vi "CRYO_MASTER_temp_0911.vi"() -> ()   [LabVIEW 2017]
uses:
  LSI218Data.lvclass
  LSI336Data.lvclass
  USBData.lvclass
  6240AData.lvclass
  <vilib>/Analysis/3filter.llb/FIR Filter (DBL).vi
  <vilib>/DAQmx/create/channels.llb/DAQmx Create Channel (DO-Digital Output).vi
  <vilib>/DAQmx/miscellaneous.llb/DAQmx Fill In Error Info.vi
  <vilib>/DAQmx/create/channels.llb/DAQmx Create Channel (AO-Voltage-Basic).vi
  <vilib>/Analysis/NI_AALBase.lvlib
panel:
  in  "Record interval":i64=10
  out "Cycle #":u32=18
  in  "Measurement Interval (s)":dbl=1.0
  in  "Stop Button":bool
  in  "?":T1(tab)
  out "error out (USB6210/6218 AOUT)":errorcluster
  in  "AOUT 1 Label":string="KIKUSUI_I"
  in  "AOUT 0 Label":string="KIKUSUI_V"
  in  "DOUT Labels":string[](array[string])=["V1_NO", "V2_NC", "CV1"]
  in  "AOUT for Current CTRL":tag="Dev1/ao1"
  in  "AOUT For Voltage CTRL":tag="Dev1/ao0"
  out "AO task out":refnum<k21>="20200910_155539_AO"
  in  "Analog Out ON?":bool
  in  "InstName (USB6218)":string="USB6218"
  in  "USB6218 Config":T2(array[cluster])=[{"Label"="F_1", "FileFormat"="%5.5f", "Active?"=TRUE, "Physical CH"="Dev1/ai0", " terminal\n type"=10083, "ConversionType"={"Type"=enum."SimpleProp", "ConversionParameters"=[0.0, 5.0, 0.0, 500.0]}, "VoltageLimits"=[0.0, 5.0]}, {"Label"="F_2", "FileFormat"="%5.5f", "Active?"=TRUE, "Physical CH"="Dev1/ai1", " terminal\n type"=10083, "ConversionType"={"Type"=enum."SimpleProp", "ConversionParameters"=[0.0, 5.0, 0.0, 200.0]}, "VoltageLimits"=[0.0, 5.0]}, {"Label"="F_3", "FileFormat"="%5.5f", "Active?"=TRUE, "Physical CH"="Dev1/ai2", " terminal\n type"=10083, "ConversionType"={"Type"=enum."SimpleProp", "ConversionParameters"=[0.0, 5.0, 0.0, 200.0]}, "VoltageLimits"=[0.0, 5.0]}, {"Label"="F_4", "FileFormat"="%5.5f", "Active?"=TRUE, "Physical CH"="Dev1/ai3", " terminal\n type"=10083, "ConversionType"={"Type"=enum."SimpleProp", "ConversionParameters"=[0.0, 5.0, 0.0, 500.0]}, "VoltageLimits"=[0.0, 5.0]}, {"Label"="F_5", "FileFormat"="%5.5f", "Active?"=TRUE, "Physical CH"="Dev1/ai4", " terminal\n type"=10083, "ConversionType"={"Type"=enum."SimpleProp", "ConversionParameters"=[0.0, 5.0, 0.0, 500.0]}, "VoltageLimits"=[0.0, 5.0]}, {"Label"="I_CV", "FileFormat"="%3.5f", "Active?"=FALSE, "Physical CH"="Dev1/ai5", " terminal\n type"=10083, "ConversionType"={"Type"=enum."SimpleProp", "ConversionParameters"=[0.0, 5.0, 0.0, 2000.0]}, "VoltageLimits"=[0.0, 5.0]}, {"Label"="CV1_answer", "FileFormat"="%3.5f", "Active?"=FALSE, "Physical CH"="Dev1/ai6", " terminal\n type"=10083, "ConversionType"={"Type"=enum."Raw", "ConversionParameters"=[]}, "VoltageLimits"=[]}] {"terminal\n type" items=["Default"=-1, "RSE"=10083, "NRSE"=10078, "Differential"=10106, "Pseudodifferential"=12529]}
  out "error out (USB6218)":errorcluster={"status"=TRUE, "code"=-200489, "source"="DAQmx Create Channel (AI-Voltage-Basic).vi:1780001<append>\n<B>Channel Name: </B>Dev1/ai2\n\n<B>Task Name: </B>PreCooling_20200910_155626_USB6218__AIN"}
  out "error out (USB6210/6218 DOUT)":errorcluster
  out "Target Index":i32=6
  out "DOUT task out":refnum<k21>="20200910_155626_DO"
  in  "DOUT Physical CH":tag[](array[tag])=["Dev1/port1/line0", "Dev1/port1/line1", "Dev1/port1/line2"]
  in  "Dewar Regularization \nTarget Signal Label":string="P_Dewar"
  in  "Digital Out ON?":bool=TRUE
  in  "USB6210 Config":T2(array[cluster])=[{"Label"="P_ins", "FileFormat"="%5.5e", "Active?"=TRUE, "Physical CH"="Dev2/ai0", " terminal\n type"=10083, "ConversionType"={"Type"=enum."CC-10_LOG", "ConversionParameters"=[0.5, 9.0, 0.0, 1.0]}, "VoltageLimits"=[0.0, 10.0]}, {"Label"="P_4Kres", "FileFormat"="%5.5e", "Active?"=TRUE, "Physical CH"="Dev2/ai1", " terminal\n type"=10083, "ConversionType"={"Type"=enum."SimpleProp", "ConversionParameters"=[1.0, 5.0, 0.0, 200000.0]}, "VoltageLimits"=[0.0, 5.0]}, {"Label"="P_3HeIN", "FileFormat"="%5.5e", "Active?"=TRUE, "Physical CH"="Dev2/ai2", " terminal\n type"=10083, "ConversionType"={"Type"=enum."SimpleProp", "ConversionParameters"=[1.0, 5.0, 0.0, 200000.0]}, "VoltageLimits"=[0.0, 5.0]}, {"Label"="P_SldRTN", "FileFormat"="%5.5e", "Active?"=TRUE, "Physical CH"="Dev2/ai3", " terminal\n type"=10083, "ConversionType"={"Type"=enum."SimpleProp", "ConversionParameters"=[1.0, 5.0, 0.0, 200000.0]}, "VoltageLimits"=[0.0, 5.0]}, {"Label"="P_3Hepot", "FileFormat"="%5.5e", "Active?"=TRUE, "Physical CH"="Dev2/ai4", " terminal\n type"=10083, "ConversionType"={"Type"=enum."SimpleProp", "ConversionParameters"=[0.0, 10.0, 0.0, 133320.0]}, "VoltageLimits"=[0.0, 10.0]}, {"Label"="P_1Kpot", "FileFormat"="%5.5e", "Active?"=TRUE, "Physical CH"="Dev2/ai5", " terminal\n type"=10083, "ConversionType"={"Type"=enum."SimpleProp", "ConversionParameters"=[0.0, 10.0, 0.0, 133320.0]}, "VoltageLimits"=[0.0, 10.0]}, {"Label"="P_Dewar", "FileFormat"="%5.5e", "Active?"=TRUE, "Physical CH"="Dev2/ai6", " terminal\n type"=10083, "ConversionType"={"Type"=enum."SimpleProp", "ConversionParameters"=[1.0, 5.0, 0.0, 200000.0]}, "VoltageLimits"=[0.0, 5.0]}, {"Label"="DP_HEX4", "FileFormat"="%5.5e", "Active?"=TRUE, "Physical CH"="Dev2/ai7", " terminal\n type"=10083, "ConversionType"={"Type"=enum."SimpleProp", "ConversionParameters"=[1.0, 5.0, 0.0, 1000.0]}, "VoltageLimits"=[0.0, 5.0]}, {"Label"="DP_HEX5", "FileFormat"="%5.5e", "Active?"=TRUE, "Physical CH"="Dev2/ai8", " terminal\n type"=10083, "ConversionType"={"Type"=enum."SimpleProp", "ConversionParameters"=[1.0, 5.0, 0.0, 20000.0]}, "VoltageLimits"=[0.0, 5.0]}, {"Label"="L1", "FileFormat"="%5.5f", "Active?"=TRUE, "Physical CH"="Dev2/ai9", " terminal\n type"=10083, "ConversionType"={"Type"=enum."SimpleProp", "ConversionParameters"=[0.0, 10.0, 0.0, 100.0]}, "VoltageLimits"=[0.0, 10.0]}, {"Label"="L2-1", "FileFormat"="%5.5f", "Active?"=TRUE, "Physical CH"="Dev2/ai10", " terminal\n type"=10083, "ConversionType"={"Type"=enum."SimpleProp", "ConversionParameters"=[0.0, 10.0, 0.0, 100.0]}, "VoltageLimits"=[0.0, 10.0]}, {"Label"="L2-2", "FileFormat"="%5.5f", "Active?"=TRUE, "Physical CH"="Dev2/ai11", " terminal\n type"=10083, "ConversionType"={"Type"=enum."SimpleProp", "ConversionParameters"=[0.0, 10.0, 0.0, 100.0]}, "VoltageLimits"=[0.0, 10.0]}, {"Label"="L3", "FileFormat"="%5.5f", "Active?"=TRUE, "Physical CH"="Dev2/ai12", " terminal\n type"=10083, "ConversionType"={"Type"=enum."SimpleProp", "ConversionParameters"=[0.0, 10.0, 0.0, 100.0]}, "VoltageLimits"=[0.0, 10.0]}] {"terminal\n type" items=["Default"=-1, "RSE"=10083, "NRSE"=10078, "Differential"=10106, "Pseudodifferential"=12529]}
  in  "RUN identifier":string="PreCooling"
  in  "Base Path":path=path "C:/LabVIEW/DATA/Precooling"
  in  "InstName (USB6210)":string="USB6210"
  out "error out (USB6210)":errorcluster
  out "File Refn USB AO":refnum<file>
  out "File Refn USB DO":refnum<file>
  out "error out (LSI336)":errorcluster
  in  "InstName (LSI336)":string="LSI336"
  in  "FileFormat (336)":string="%4.4f"
  in  "LSI336Settings(X,Y)":T3(array[cluster])=[{"LSIName"="LSi336X", "Labels"=["T1K3-1", "T1K3-2", "T3He5", "T3He8"], "SensorLocations"=[enum."T1K3-1", enum."T1K3-2", enum."T3He5", enum."T3He8"], "Active?"=TRUE, "VISA res. name"="GPIB0::6::INSTR"}, {"LSIName"="LSi336Y", "Labels"=["T3He6-1", "T3He6-2", "T3He7-1", "T3He7-2"], "SensorLocations"=[enum."T3He6-1", enum."T3He6-2", enum."T3He7-1", enum."T3He7-2"], "Active?"=TRUE, "VISA res. name"="GPIB0::2::INSTR"}]
  in  "FileFormat (218)":string="%4.4f"
  in  "InstName (LSI218)":string="LSI218"
  in  "LSI218Settings(A-F)":T3(array[cluster])=[{"LSIName"="LSI218A", "Labels"=["T3He10", "T3He1-1", "TTH3", "TTH4", "TTH1", "TTH2", "T4He1", "T1K1"], "SensorLocations"=[enum."T3He10", enum."T3He1-1", enum."TTH3", enum."TTH4", enum."TTH1", enum."TTH2", enum."T4He1", enum."T1K1"], "Active?"=TRUE, "VISA res. name"="GPIB0::7::INSTR"}, {"LSIName"="LSI218B", "Labels"=["N.C.", "N.C.", "N.C.", "N.C.", "T3He2-1", "T3He2-2", "T3He3", "T3He1-4"], "SensorLocations"=[enum."N.C.", enum."N.C.", enum."N.C.", enum."T3He1-4", enum."T3He2-1", enum."T3He2-2", enum."T3He3", enum."T3He1-4"], "Active?"=TRUE, "VISA res. name"="GPIB0::4::INSTR"}, {"LSIName"="LSI218C", "Labels"=["T4He3-1", "T4He3-2", "T4He3-3", "T4He3-4", "T4He2-1", "T4He2-2", "T4He4", "T4He5"], "SensorLocations"=[enum."T4He3-1", enum."T4He3-2", enum."T4He3-3", enum."T4He3-4", enum."T4He2-1", enum."T4He2-2", enum."T4He4", enum."T4He5"], "Active?"=TRUE, "VISA res. name"="GPIB0::3::INSTR"}, {"LSIName"="LSI218D", "Labels"=["T4He6", "T4He9", "T3He1-2", "T3He1-3", "T4He7", "T4He8", "T4He10", "T1K6"], "SensorLocations"=[enum."T4He6", enum."T4He9", enum."T3He1-2", enum."T3He1-3", enum."T4He7", enum."T4He8", enum."T4He10", enum."T1K6"], "Active?"=TRUE, "VISA res. name"="GPIB0::5::INSTR"}, {"LSIName"="LSI218E", "Labels"=["TIP1", "N.C.", "TIP2", "N.C.", "TIP3", "TIP4", "TIP5", "N.C."], "SensorLocations"=[enum."TIP1", enum."N.C.", enum."TIP2", enum."N.C.", enum."TIP3", enum."TIP4", enum."TIP5", enum."N.C."], "Active?"=TRUE, "VISA res. name"="GPIB0::11::INSTR"}, {"LSIName"="LSI218F", "Labels"=["T1K2", "T1K4", "T1K5", "T3He4", "T3He9", "TIP6", "N.C.", "N.C."], "SensorLocations"=[enum."T1K2", enum."T1K4", enum."T1K5", enum."T3He4", enum."T3He9", enum."TIP6", enum."N.C.", enum."N.C."], "Active?"=TRUE, "VISA res. name"="GPIB0::8::INSTR"}]
  out "error out (LSI218)":errorcluster
  in  "FIle suffix 4":string="Graph4"
  in  "Take Screenshot! 4":bool
  in  "FIle suffix 3":string="Graph3"
  in  "Take Screenshot! 3":bool
  in  "FIle suffix 2":string="Graph2"
  in  "Take Screenshot! 2":bool
  in  "FIle suffix 1":string="Graph1"
  in  "Take Screenshot! 1":bool
  in  "log/linear 2":bool
  in  "Tab Control 2":T4(tab)=enum."USB6218"
  in  "Plot selecter (USB6210)\n    1      2     3     4":bool[][](array[boolean])=[[FALSE, FALSE, TRUE, FALSE], [FALSE, FALSE, TRUE, FALSE], [FALSE, FALSE, TRUE, FALSE], [FALSE, FALSE, TRUE, FALSE], [FALSE, FALSE, TRUE, FALSE], [FALSE, FALSE, TRUE, FALSE], [TRUE, FALSE, FALSE, FALSE], [FALSE, FALSE, TRUE, FALSE], [FALSE, FALSE, TRUE, FALSE], [FALSE, FALSE, FALSE, TRUE], [FALSE, FALSE, FALSE, TRUE], [FALSE, FALSE, FALSE, TRUE], [FALSE, FALSE, FALSE, TRUE], [FALSE, FALSE, FALSE, FALSE], [FALSE, FALSE, FALSE, FALSE], [FALSE, FALSE, FALSE, FALSE]]
  out "All Labels (USB6210)":string[](array[string])=["P_ins", "P_4Kres", "P_3HeIN", "P_SldRTN", "P_3Hepot", "P_1Kpot", "P_Dewar", "DP_HEX4", "DP_HEX5", "L1", "L2-1", "L2-2", "L3"]
  out "Last Data \n(USB6210)":dbl[](array[numeric])=[0.0009060437653636275, 100884.97913376133, 100585.6935800327, 100396.58457551748, 100537.343311204, 100655.70674054678, 101557.55033670987, -10.021506447432133, 71.06102831736294, 100.09004251119043, 0.10469622427214367, 0.11521822711602545, 99.57181211647702] format="%#_6e"
  out "Time of Last Measurement (USB6210)":timestamp=timestamp(3682565805.197301 s since 1904-01-01)
  out "USB6210 Status":T5(ring)=enum."Ready"
  out "Last Vol\n(USB6210)":dbl[](array[numeric])=[5.978574588130271, 3.0176995826752266, 3.011713871600654, 3.0079316915103496, 7.541054853825682, 7.549932998840893, 3.0311510067341976, 0.9599139742102715, 1.0142122056634726, 10.009004251119043, 0.010469622427214368, 0.011521822711602545, 9.957181211647702] format="%_5f"
  out "Time of Last Measurement (USB6218)":timestamp
  out "USB6218 Status":T5(ring)=enum."Ready"
  out "Last Vol \n(USB6218)":dbl[](array[numeric]) format="%_5f"
  out "Last Data \n(USB6218)":dbl[](array[numeric]) format="%#_6e"
  out "All Labels (USB6218)":string[](array[string])
  in  "Plot selecter (USB6218)\n    1      2     3     4":bool[][](array[boolean])=[[FALSE, FALSE, TRUE, FALSE], [FALSE, FALSE, TRUE, FALSE], [FALSE, FALSE, TRUE, FALSE], [FALSE, FALSE, TRUE, FALSE], [FALSE, FALSE, TRUE, FALSE], [FALSE, FALSE, TRUE, FALSE], [TRUE, FALSE, FALSE, FALSE], [FALSE, FALSE, TRUE, FALSE], [FALSE, FALSE, TRUE, FALSE], [FALSE, FALSE, FALSE, TRUE], [FALSE, FALSE, FALSE, TRUE], [FALSE, FALSE, FALSE, TRUE], [FALSE, FALSE, FALSE, TRUE], [FALSE, FALSE, FALSE, FALSE], [FALSE, FALSE, FALSE, FALSE], [FALSE, FALSE, FALSE, FALSE]]
  out "Time of Last Measurement (LSI218)":timestamp=timestamp(3682565805.197301 s since 1904-01-01)
  out "LSI218 Status":T6(ring)=enum."Measuring"
  out "Last Data \nLSI218 (1)":dbl[](array[numeric])=[297.63, 297.76, 296.71, 297.24, 295.38, 295.52, 294.91, 295.07, 30.0, 0.0, 0.0, 0.0, 296.58, 296.99, 295.68, 297.19, 297.39, 297.55, 297.28, 297.31, 296.61, 296.28, 296.32, 296.17]
  out "Labels LSI218 (1)":string[](array[string])=["T3He10", "T3He1-1", "TTH3", "TTH4", "TTH1", "TTH2", "T4He1", "T1K1", "N.C.", "N.C.", "N.C.", "N.C.", "T3He2-1", "T3He2-2", "T3He3", "T3He1-4", "T4He3-1", "T4He3-2", "T4He3-3", "T4He3-4", "T4He2-1", "T4He2-2", "T4He4", "T4He5"]
  in  "Plot selecter LSI218(1)\n    1      2     3     4":bool[][](array[boolean])=[[FALSE, FALSE, FALSE, FALSE], [FALSE, FALSE, FALSE, FALSE], [FALSE, FALSE, FALSE, FALSE], [FALSE, FALSE, FALSE, FALSE], [FALSE, FALSE, FALSE, FALSE], [FALSE, FALSE, FALSE, FALSE], [FALSE, FALSE, FALSE, FALSE], [FALSE, FALSE, FALSE, FALSE], [FALSE, FALSE, FALSE, FALSE], [FALSE, FALSE, FALSE, FALSE], [FALSE, FALSE, FALSE, FALSE], [FALSE, FALSE, FALSE, FALSE], [FALSE, FALSE, FALSE, FALSE], [FALSE, FALSE, FALSE, FALSE], [FALSE, FALSE, FALSE, FALSE], [FALSE, FALSE, FALSE, FALSE], [FALSE, FALSE, FALSE, FALSE], [FALSE, FALSE, FALSE, FALSE], [FALSE, FALSE, FALSE, FALSE], [FALSE, FALSE, FALSE, FALSE], [FALSE, FALSE, FALSE, FALSE], [FALSE, FALSE, FALSE, FALSE], [FALSE, FALSE, FALSE, FALSE], [FALSE, FALSE, FALSE, FALSE]]
  out "Active?\n (1)":bool[](array[boolean])=[TRUE, TRUE, TRUE, TRUE, TRUE, TRUE, TRUE, TRUE, TRUE, TRUE, TRUE, TRUE, TRUE, TRUE, TRUE, TRUE, TRUE, TRUE, TRUE, TRUE, TRUE, TRUE, TRUE, TRUE]
  out "Labels LSI218 (2)":string[](array[string])=["T4He6", "T4He9", "T3He1-2", "T3He1-3", "T4He7", "T4He8", "T4He10", "T1K6", "TIP1", "N.C.", "TIP2", "N.C.", "TIP3", "TIP4", "TIP5", "N.C.", "T1K2", "T1K4", "T1K5", "T3He4", "T3He9", "TIP6", "N.C.", "N.C."]
  out "Active?\n(2)":bool[](array[boolean])=[TRUE, TRUE, TRUE, TRUE, TRUE, TRUE, TRUE, TRUE, TRUE, TRUE, TRUE, TRUE, TRUE, TRUE, TRUE, TRUE, TRUE, TRUE, TRUE, TRUE, TRUE, TRUE, TRUE, TRUE]
  out "Last Data \nLSI218 (2)":dbl[](array[numeric])=[296.4, 297.17, 297.92, 297.51, 296.71, 297.02, 296.96, 297.42, 296.77, 0.0, 296.31, 688.49, 296.06, 295.63, 295.73, 688.58, 302.11, 301.08, 296.91, 291.77, 288.69, 280.14, 0.433, 0.0]
  in  "Plot selecter LSI218(2)\n    1      2     3     4":bool[][](array[boolean])=[[FALSE, TRUE, FALSE, FALSE], [FALSE, TRUE, FALSE, FALSE], [FALSE, TRUE, FALSE, FALSE], [FALSE, TRUE, FALSE, FALSE], [FALSE, TRUE, FALSE, FALSE], [FALSE, TRUE, FALSE, FALSE], [FALSE, TRUE, FALSE, FALSE], [FALSE, TRUE, FALSE, FALSE], [FALSE, TRUE, FALSE, FALSE], [FALSE, TRUE, FALSE, FALSE], [FALSE, TRUE, FALSE, FALSE], [FALSE, FALSE, FALSE, FALSE], [FALSE, FALSE, FALSE, FALSE], [FALSE, FALSE, FALSE, FALSE], [FALSE, FALSE, FALSE, FALSE], [FALSE, FALSE, FALSE, FALSE], [FALSE, FALSE, FALSE, FALSE], [FALSE, FALSE, FALSE, FALSE], [FALSE, FALSE, FALSE, FALSE], [FALSE, FALSE, FALSE, FALSE], [FALSE, FALSE, FALSE, FALSE], [FALSE, FALSE, FALSE, FALSE], [FALSE, FALSE, FALSE, FALSE], [FALSE, FALSE, FALSE, FALSE]]
  in  "Plot selecter LSI336 \n     1      2     3     4":bool[][](array[boolean])=[[FALSE, TRUE, FALSE, FALSE], [FALSE, TRUE, FALSE, FALSE], [FALSE, TRUE, FALSE, FALSE], [FALSE, TRUE, FALSE, FALSE], [FALSE, TRUE, FALSE, FALSE], [FALSE, TRUE, FALSE, FALSE], [FALSE, TRUE, FALSE, FALSE], [FALSE, TRUE, FALSE, FALSE]]
  out "Time of Last Measurement (LSI336) 2":timestamp=timestamp(3682565805.197301 s since 1904-01-01)
  out "Last Data \nLSI336":dbl[](array[numeric])=[296.838, 296.434, 296.022, 296.217, 295.887, 295.842, 295.916, 296.504]
  out "Active?\n(LSI336)":bool[](array[boolean])=[TRUE, TRUE, TRUE, TRUE, TRUE, TRUE, TRUE, TRUE]
  out "Labels LSI336":string[](array[string])=["T1K3-1", "T1K3-2", "T3He5", "T3He8", "T3He6-1", "T3He6-2", "T3He7-1", "T3He7-2"]
  out "LSI336 Status":T6(ring)=enum."Measuring"
  out "Graph 1":T7(graph)=[{"TimeArray"=[timestamp(3682565788.1889906 s since 1904-01-01), timestamp(3682565789.190164 s since 1904-01-01), timestamp(3682565790.191844 s since 1904-01-01), timestamp(3682565791.191016 s since 1904-01-01), timestamp(3682565792.191493 s since 1904-01-01), timestamp(3682565793.190962 s since 1904-01-01), timestamp(3682565794.192923 s since 1904-01-01), timestamp(3682565795.1943216 s since 1904-01-01), timestamp(3682565796.1945167 s since 1904-01-01), timestamp(3682565797.194023 s since 1904-01-01), timestamp(3682565798.195678 s since 1904-01-01), timestamp(3682565799.194545 s since 1904-01-01), timestamp(3682565800.194017 s since 1904-01-01), timestamp(3682565801.196416 s since 1904-01-01), timestamp(3682565802.1962314 s since 1904-01-01), timestamp(3682565803.1960993 s since 1904-01-01), timestamp(3682565804.196091 s since 1904-01-01), timestamp(3682565805.197301 s since 1904-01-01)], "LDArray"=[98878.77979362432]}] caption="XY Graph"
  in  "log/linear 1":bool
  out "Graph 2":T8(graph)=[{"TimeArray"=[timestamp(3682565788.1889906 s since 1904-01-01), timestamp(3682565789.190164 s since 1904-01-01), timestamp(3682565790.191844 s since 1904-01-01), timestamp(3682565791.191016 s since 1904-01-01), timestamp(3682565792.191493 s since 1904-01-01), timestamp(3682565793.190962 s since 1904-01-01), timestamp(3682565794.192923 s since 1904-01-01), timestamp(3682565795.1943216 s since 1904-01-01), timestamp(3682565796.1945167 s since 1904-01-01), timestamp(3682565797.194023 s since 1904-01-01), timestamp(3682565798.1947985 s since 1904-01-01), timestamp(3682565799.194545 s since 1904-01-01), timestamp(3682565800.194017 s since 1904-01-01), timestamp(3682565801.1955366 s since 1904-01-01), timestamp(3682565802.1962314 s since 1904-01-01), timestamp(3682565803.1960993 s since 1904-01-01), timestamp(3682565804.196091 s since 1904-01-01), timestamp(3682565805.197301 s since 1904-01-01)], "DataArray"=[296.44, 296.4, 296.4, 296.4, 296.43, 296.43, 296.39, 296.41, 296.43, 296.4, 296.39, 296.41, 296.38, 296.38, 296.41, 296.42, 296.41, 296.4]}, {"TimeArray"=[timestamp(3682565788.1889906 s since 1904-01-01), timestamp(3682565789.190164 s since 1904-01-01), timestamp(3682565790.191844 s since 1904-01-01), timestamp(3682565791.191016 s since 1904-01-01), timestamp(3682565792.191493 s since 1904-01-01), timestamp(3682565793.190962 s since 1904-01-01), timestamp(3682565794.192923 s since 1904-01-01), timestamp(3682565795.1943216 s since 1904-01-01), timestamp(3682565796.1945167 s since 1904-01-01), timestamp(3682565797.194023 s since 1904-01-01), timestamp(3682565798.1947985 s since 1904-01-01), timestamp(3682565799.194545 s since 1904-01-01), timestamp(3682565800.194017 s since 1904-01-01), timestamp(3682565801.1955366 s since 1904-01-01), timestamp(3682565802.1962314 s since 1904-01-01), timestamp(3682565803.1960993 s since 1904-01-01), timestamp(3682565804.196091 s since 1904-01-01), timestamp(3682565805.197301 s since 1904-01-01)], "DataArray"=[297.15, 297.15, 297.15, 297.15, 297.16, 297.16, 297.14, 297.14, 297.15, 297.13, 297.16, 297.14, 297.14, 297.14, 297.12, 297.14, 297.14, 297.17]}, {"TimeArray"=[timestamp(3682565788.1889906 s since 1904-01-01), timestamp(3682565789.190164 s since 1904-01-01), timestamp(3682565790.191844 s since 1904-01-01), timestamp(3682565791.191016 s since 1904-01-01), timestamp(3682565792.191493 s since 1904-01-01), timestamp(3682565793.190962 s since 1904-01-01), timestamp(3682565794.192923 s since 1904-01-01), timestamp(3682565795.1943216 s since 1904-01-01), timestamp(3682565796.1945167 s since 1904-01-01), timestamp(3682565797.194023 s since 1904-01-01), timestamp(3682565798.1947985 s since 1904-01-01), timestamp(3682565799.194545 s since 1904-01-01), timestamp(3682565800.194017 s since 1904-01-01), timestamp(3682565801.1955366 s since 1904-01-01), timestamp(3682565802.1962314 s since 1904-01-01), timestamp(3682565803.1960993 s since 1904-01-01), timestamp(3682565804.196091 s since 1904-01-01), timestamp(3682565805.197301 s since 1904-01-01)], "DataArray"=[297.94, 297.93, 297.96, 297.92, 297.94, 297.93, 297.93, 297.93, 297.93, 297.94, 297.96, 297.93, 297.93, 297.94, 297.93, 297.93, 297.93, 297.92]}, {"TimeArray"=[timestamp(3682565788.1889906 s since 1904-01-01), timestamp(3682565789.190164 s since 1904-01-01), timestamp(3682565790.191844 s since 1904-01-01), timestamp(3682565791.191016 s since 1904-01-01), timestamp(3682565792.191493 s since 1904-01-01), timestamp(3682565793.190962 s since 1904-01-01), timestamp(3682565794.192923 s since 1904-01-01), timestamp(3682565795.1943216 s since 1904-01-01), timestamp(3682565796.1945167 s since 1904-01-01), timestamp(3682565797.194023 s since 1904-01-01), timestamp(3682565798.1947985 s since 1904-01-01), timestamp(3682565799.194545 s since 1904-01-01), timestamp(3682565800.194017 s since 1904-01-01), timestamp(3682565801.1955366 s since 1904-01-01), timestamp(3682565802.1962314 s since 1904-01-01), timestamp(3682565803.1960993 s since 1904-01-01), timestamp(3682565804.196091 s since 1904-01-01), timestamp(3682565805.197301 s since 1904-01-01)], "DataArray"=[297.53, 297.5, 297.52, 297.51, 297.52, 297.52, 297.54, 297.54, 297.53, 297.51, 297.52, 297.52, 297.53, 297.52, 297.53, 297.52, 297.53, 297.51]}, {"TimeArray"=[timestamp(3682565788.1889906 s since 1904-01-01), timestamp(3682565789.190164 s since 1904-01-01), timestamp(3682565790.191844 s since 1904-01-01), timestamp(3682565791.191016 s since 1904-01-01), timestamp(3682565792.191493 s since 1904-01-01), timestamp(3682565793.190962 s since 1904-01-01), timestamp(3682565794.192923 s since 1904-01-01), timestamp(3682565795.1943216 s since 1904-01-01), timestamp(3682565796.1945167 s since 1904-01-01), timestamp(3682565797.194023 s since 1904-01-01), timestamp(3682565798.1947985 s since 1904-01-01), timestamp(3682565799.194545 s since 1904-01-01), timestamp(3682565800.194017 s since 1904-01-01), timestamp(3682565801.1955366 s since 1904-01-01), timestamp(3682565802.1962314 s since 1904-01-01), timestamp(3682565803.1960993 s since 1904-01-01), timestamp(3682565804.196091 s since 1904-01-01), timestamp(3682565805.197301 s since 1904-01-01)], "DataArray"=[296.7, 296.71, 296.71, 296.72, 296.7, 296.69, 296.7, 296.69, 296.7, 296.7, 296.7, 296.7, 296.71, 296.7, 296.71, 296.68, 296.7, 296.71]}, {"TimeArray"=[timestamp(3682565788.1889906 s since 1904-01-01), timestamp(3682565789.190164 s since 1904-01-01), timestamp(3682565790.191844 s since 1904-01-01), timestamp(3682565791.191016 s since 1904-01-01), timestamp(3682565792.191493 s since 1904-01-01), timestamp(3682565793.190962 s since 1904-01-01), timestamp(3682565794.192923 s since 1904-01-01), timestamp(3682565795.1943216 s since 1904-01-01), timestamp(3682565796.1945167 s since 1904-01-01), timestamp(3682565797.194023 s since 1904-01-01), timestamp(3682565798.1947985 s since 1904-01-01), timestamp(3682565799.194545 s since 1904-01-01), timestamp(3682565800.194017 s since 1904-01-01), timestamp(3682565801.1955366 s since 1904-01-01), timestamp(3682565802.1962314 s since 1904-01-01), timestamp(3682565803.1960993 s since 1904-01-01), timestamp(3682565804.196091 s since 1904-01-01), timestamp(3682565805.197301 s since 1904-01-01)], "DataArray"=[297.02, 297.03, 297.04, 297.03, 297.0, 297.02, 297.0, 297.02, 297.05, 297.0, 297.0, 297.0, 297.01, 297.02, 297.03, 297.0, 297.02, 297.02]}, {"TimeArray"=[timestamp(3682565788.1889906 s since 1904-01-01), timestamp(3682565789.190164 s since 1904-01-01), timestamp(3682565790.191844 s since 1904-01-01), timestamp(3682565791.191016 s since 1904-01-01), timestamp(3682565792.191493 s since 1904-01-01), timestamp(3682565793.190962 s since 1904-01-01), timestamp(3682565794.192923 s since 1904-01-01), timestamp(3682565795.1943216 s since 1904-01-01), timestamp(3682565796.1945167 s since 1904-01-01), timestamp(3682565797.194023 s since 1904-01-01), timestamp(3682565798.1947985 s since 1904-01-01), timestamp(3682565799.194545 s since 1904-01-01), timestamp(3682565800.194017 s since 1904-01-01), timestamp(3682565801.1955366 s since 1904-01-01), timestamp(3682565802.1962314 s since 1904-01-01), timestamp(3682565803.1960993 s since 1904-01-01), timestamp(3682565804.196091 s since 1904-01-01), timestamp(3682565805.197301 s since 1904-01-01)], "DataArray"=[296.96, 296.97, 296.96, 296.98, 296.96, 296.95, 296.98, 296.99, 296.97, 296.96, 296.95, 296.94, 296.95, 296.95, 296.97, 296.95, 296.96, 296.96]}, {"TimeArray"=[timestamp(3682565788.1889906 s since 1904-01-01), timestamp(3682565789.190164 s since 1904-01-01), timestamp(3682565790.191844 s since 1904-01-01), timestamp(3682565791.191016 s since 1904-01-01), timestamp(3682565792.191493 s since 1904-01-01), timestamp(3682565793.190962 s since 1904-01-01), timestamp(3682565794.192923 s since 1904-01-01), timestamp(3682565795.1943216 s since 1904-01-01), timestamp(3682565796.1945167 s since 1904-01-01), timestamp(3682565797.194023 s since 1904-01-01), timestamp(3682565798.1947985 s since 1904-01-01), timestamp(3682565799.194545 s since 1904-01-01), timestamp(3682565800.194017 s since 1904-01-01), timestamp(3682565801.1955366 s since 1904-01-01), timestamp(3682565802.1962314 s since 1904-01-01), timestamp(3682565803.1960993 s since 1904-01-01), timestamp(3682565804.196091 s since 1904-01-01), timestamp(3682565805.197301 s since 1904-01-01)], "DataArray"=[297.4, 297.41, 297.4, 297.4, 297.41, 297.42, 297.41, 297.42, 297.41, 297.4, 297.42, 297.41, 297.42, 297.39, 297.42, 297.4, 297.42, 297.42]}, {"TimeArray"=[timestamp(3682565788.1889906 s since 1904-01-01), timestamp(3682565789.190164 s since 1904-01-01), timestamp(3682565790.191844 s since 1904-01-01), timestamp(3682565791.191016 s since 1904-01-01), timestamp(3682565792.191493 s since 1904-01-01), timestamp(3682565793.190962 s since 1904-01-01), timestamp(3682565794.192923 s since 1904-01-01), timestamp(3682565795.1943216 s since 1904-01-01), timestamp(3682565796.1945167 s since 1904-01-01), timestamp(3682565797.194023 s since 1904-01-01), timestamp(3682565798.1947985 s since 1904-01-01), timestamp(3682565799.194545 s since 1904-01-01), timestamp(3682565800.194017 s since 1904-01-01), timestamp(3682565801.1955366 s since 1904-01-01), timestamp(3682565802.1962314 s since 1904-01-01), timestamp(3682565803.1960993 s since 1904-01-01), timestamp(3682565804.196091 s since 1904-01-01), timestamp(3682565805.197301 s since 1904-01-01)], "DataArray"=[296.76, 296.76, 296.76, 296.76, 296.76, 296.77, 296.76, 296.77, 296.76, 296.76, 296.76, 296.76, 296.76, 296.76, 296.76, 296.76, 296.77, 296.77]}, {"TimeArray"=[timestamp(3682565788.1889906 s since 1904-01-01), timestamp(3682565789.190164 s since 1904-01-01), timestamp(3682565790.191844 s since 1904-01-01), timestamp(3682565791.191016 s since 1904-01-01), timestamp(3682565792.191493 s since 1904-01-01), timestamp(3682565793.190962 s since 1904-01-01), timestamp(3682565794.192923 s since 1904-01-01), timestamp(3682565795.1943216 s since 1904-01-01), timestamp(3682565796.1945167 s since 1904-01-01), timestamp(3682565797.194023 s since 1904-01-01), timestamp(3682565798.1947985 s since 1904-01-01), timestamp(3682565799.194545 s since 1904-01-01), timestamp(3682565800.194017 s since 1904-01-01), timestamp(3682565801.1955366 s since 1904-01-01), timestamp(3682565802.1962314 s since 1904-01-01), timestamp(3682565803.1960993 s since 1904-01-01), timestamp(3682565804.196091 s since 1904-01-01), timestamp(3682565805.197301 s since 1904-01-01)], "DataArray"=[0.0, 0.0, 0.0, 0.0, 0.0, 0.0, 0.0, 0.0, 0.0, 0.0, 0.0, 0.0, 0.0, 0.0, 0.0, 0.0, 0.0, 0.0]}, {"TimeArray"=[timestamp(3682565788.1889906 s since 1904-01-01), timestamp(3682565789.190164 s since 1904-01-01), timestamp(3682565790.191844 s since 1904-01-01), timestamp(3682565791.191016 s since 1904-01-01), timestamp(3682565792.191493 s since 1904-01-01), timestamp(3682565793.190962 s since 1904-01-01), timestamp(3682565794.192923 s since 1904-01-01), timestamp(3682565795.1943216 s since 1904-01-01), timestamp(3682565796.1945167 s since 1904-01-01), timestamp(3682565797.194023 s since 1904-01-01), timestamp(3682565798.1947985 s since 1904-01-01), timestamp(3682565799.194545 s since 1904-01-01), timestamp(3682565800.194017 s since 1904-01-01), timestamp(3682565801.1955366 s since 1904-01-01), timestamp(3682565802.1962314 s since 1904-01-01), timestamp(3682565803.1960993 s since 1904-01-01), timestamp(3682565804.196091 s since 1904-01-01), timestamp(3682565805.197301 s since 1904-01-01)], "DataArray"=[296.31, 296.33, 296.32, 296.31, 296.33, 296.32, 296.32, 296.32, 296.32, 296.32, 296.33, 296.33, 296.31, 296.32, 296.33, 296.31, 296.32, 296.31]}, {"TimeArray"=[timestamp(3682565788.1889906 s since 1904-01-01), timestamp(3682565789.190164 s since 1904-01-01), timestamp(3682565790.191844 s since 1904-01-01), timestamp(3682565791.191016 s since 1904-01-01), timestamp(3682565792.191493 s since 1904-01-01), timestamp(3682565793.190962 s since 1904-01-01), timestamp(3682565794.192923 s since 1904-01-01), timestamp(3682565795.1943216 s since 1904-01-01), timestamp(3682565796.1945167 s since 1904-01-01), timestamp(3682565797.194023 s since 1904-01-01), timestamp(3682565798.1947985 s since 1904-01-01), timestamp(3682565799.194545 s since 1904-01-01), timestamp(3682565800.194017 s since 1904-01-01), timestamp(3682565801.1955366 s since 1904-01-01), timestamp(3682565802.1962314 s since 1904-01-01), timestamp(3682565803.1960993 s since 1904-01-01), timestamp(3682565804.196091 s since 1904-01-01), timestamp(3682565805.197301 s since 1904-01-01)], "DataArray"=[296.847, 296.84, 296.846, 296.853, 296.853, 296.84, 296.845, 296.857, 296.848, 296.872, 296.855, 296.849, 296.848, 296.854, 296.853, 296.859, 296.85, 296.838]}, {"TimeArray"=[timestamp(3682565788.1889906 s since 1904-01-01), timestamp(3682565789.190164 s since 1904-01-01), timestamp(3682565790.191844 s since 1904-01-01), timestamp(3682565791.191016 s since 1904-01-01), timestamp(3682565792.191493 s since 1904-01-01), timestamp(3682565793.190962 s since 1904-01-01), timestamp(3682565794.192923 s since 1904-01-01), timestamp(3682565795.1943216 s since 1904-01-01), timestamp(3682565796.1945167 s since 1904-01-01), timestamp(3682565797.194023 s since 1904-01-01), timestamp(3682565798.1947985 s since 1904-01-01), timestamp(3682565799.194545 s since 1904-01-01), timestamp(3682565800.194017 s since 1904-01-01), timestamp(3682565801.1955366 s since 1904-01-01), timestamp(3682565802.1962314 s since 1904-01-01), timestamp(3682565803.1960993 s since 1904-01-01), timestamp(3682565804.196091 s since 1904-01-01), timestamp(3682565805.197301 s since 1904-01-01)], "DataArray"=[296.447, 296.444, 296.434, 296.439, 296.434, 296.44, 296.441, 296.446, 296.444, 296.461, 296.459, 296.445, 296.453, 296.446, 296.443, 296.445, 296.445, 296.434]}, {"TimeArray"=[timestamp(3682565788.1889906 s since 1904-01-01), timestamp(3682565789.190164 s since 1904-01-01), timestamp(3682565790.191844 s since 1904-01-01), timestamp(3682565791.191016 s since 1904-01-01), timestamp(3682565792.191493 s since 1904-01-01), timestamp(3682565793.190962 s since 1904-01-01), timestamp(3682565794.192923 s since 1904-01-01), timestamp(3682565795.1943216 s since 1904-01-01), timestamp(3682565796.1945167 s since 1904-01-01), timestamp(3682565797.194023 s since 1904-01-01), timestamp(3682565798.1947985 s since 1904-01-01), timestamp(3682565799.194545 s since 1904-01-01), timestamp(3682565800.194017 s since 1904-01-01), timestamp(3682565801.1955366 s since 1904-01-01), timestamp(3682565802.1962314 s since 1904-01-01), timestamp(3682565803.1960993 s since 1904-01-01), timestamp(3682565804.196091 s since 1904-01-01), timestamp(3682565805.197301 s since 1904-01-01)], "DataArray"=[296.043, 296.016, 296.025, 296.028, 296.025, 296.018, 296.021, 296.016, 296.018, 296.027, 296.024, 296.016, 296.024, 296.014, 296.023, 296.031, 296.013, 296.022]}, {"TimeArray"=[timestamp(3682565788.1889906 s since 1904-01-01), timestamp(3682565789.190164 s since 1904-01-01), timestamp(3682565790.191844 s since 1904-01-01), timestamp(3682565791.191016 s since 1904-01-01), timestamp(3682565792.191493 s since 1904-01-01), timestamp(3682565793.190962 s since 1904-01-01), timestamp(3682565794.192923 s since 1904-01-01), timestamp(3682565795.1943216 s since 1904-01-01), timestamp(3682565796.1945167 s since 1904-01-01), timestamp(3682565797.194023 s since 1904-01-01), timestamp(3682565798.1947985 s since 1904-01-01), timestamp(3682565799.194545 s since 1904-01-01), timestamp(3682565800.194017 s since 1904-01-01), timestamp(3682565801.1955366 s since 1904-01-01), timestamp(3682565802.1962314 s since 1904-01-01), timestamp(3682565803.1960993 s since 1904-01-01), timestamp(3682565804.196091 s since 1904-01-01), timestamp(3682565805.197301 s since 1904-01-01)], "DataArray"=[296.255, 296.223, 296.212, 296.217, 296.221, 296.211, 296.215, 296.214, 296.221, 296.222, 296.22, 296.22, 296.215, 296.21, 296.215, 296.221, 296.21, 296.217]}, {"TimeArray"=[timestamp(3682565788.1889906 s since 1904-01-01), timestamp(3682565789.190164 s since 1904-01-01), timestamp(3682565790.191844 s since 1904-01-01), timestamp(3682565791.191016 s since 1904-01-01), timestamp(3682565792.191493 s since 1904-01-01), timestamp(3682565793.190962 s since 1904-01-01), timestamp(3682565794.192923 s since 1904-01-01), timestamp(3682565795.1943216 s since 1904-01-01), timestamp(3682565796.1945167 s since 1904-01-01), timestamp(3682565797.194023 s since 1904-01-01), timestamp(3682565798.1947985 s since 1904-01-01), timestamp(3682565799.194545 s since 1904-01-01), timestamp(3682565800.194017 s since 1904-01-01), timestamp(3682565801.1955366 s since 1904-01-01), timestamp(3682565802.1962314 s since 1904-01-01), timestamp(3682565803.1960993 s since 1904-01-01), timestamp(3682565804.196091 s since 1904-01-01), timestamp(3682565805.197301 s since 1904-01-01)], "DataArray"=[295.89, 295.881, 295.884, 295.884, 295.892, 295.875, 295.898, 295.88, 295.894, 295.891, 295.897, 295.894, 295.896, 295.879, 295.893, 295.894, 295.892, 295.887]}, {"TimeArray"=[timestamp(3682565788.1889906 s since 1904-01-01), timestamp(3682565789.190164 s since 1904-01-01), timestamp(3682565790.191844 s since 1904-01-01), timestamp(3682565791.191016 s since 1904-01-01), timestamp(3682565792.191493 s since 1904-01-01), timestamp(3682565793.190962 s since 1904-01-01), timestamp(3682565794.192923 s since 1904-01-01), timestamp(3682565795.1943216 s since 1904-01-01), timestamp(3682565796.1945167 s since 1904-01-01), timestamp(3682565797.194023 s since 1904-01-01), timestamp(3682565798.1947985 s since 1904-01-01), timestamp(3682565799.194545 s since 1904-01-01), timestamp(3682565800.194017 s since 1904-01-01), timestamp(3682565801.1955366 s since 1904-01-01), timestamp(3682565802.1962314 s since 1904-01-01), timestamp(3682565803.1960993 s since 1904-01-01), timestamp(3682565804.196091 s since 1904-01-01), timestamp(3682565805.197301 s since 1904-01-01)], "DataArray"=[295.848, 295.843, 295.842, 295.856, 295.851, 295.842, 295.843, 295.849, 295.851, 295.846, 295.842, 295.842, 295.842, 295.854, 295.833, 295.844, 295.852, 295.842]}, {"TimeArray"=[timestamp(3682565788.1889906 s since 1904-01-01), timestamp(3682565789.190164 s since 1904-01-01), timestamp(3682565790.191844 s since 1904-01-01), timestamp(3682565791.191016 s since 1904-01-01), timestamp(3682565792.191493 s since 1904-01-01), timestamp(3682565793.190962 s since 1904-01-01), timestamp(3682565794.192923 s since 1904-01-01), timestamp(3682565795.1943216 s since 1904-01-01), timestamp(3682565796.1945167 s since 1904-01-01), timestamp(3682565797.194023 s since 1904-01-01), timestamp(3682565798.1947985 s since 1904-01-01), timestamp(3682565799.194545 s since 1904-01-01), timestamp(3682565800.194017 s since 1904-01-01), timestamp(3682565801.1955366 s since 1904-01-01), timestamp(3682565802.1962314 s since 1904-01-01), timestamp(3682565803.1960993 s since 1904-01-01), timestamp(3682565804.196091 s since 1904-01-01), timestamp(3682565805.197301 s since 1904-01-01)], "DataArray"=[295.91, 295.913, 295.921, 295.929, 295.916, 295.915, 295.921, 295.916, 295.936, 295.917, 295.915, 295.932, 295.924, 295.919, 295.922, 295.92, 295.908, 295.916]}, {"TimeArray"=[timestamp(3682565788.1889906 s since 1904-01-01), timestamp(3682565789.190164 s since 1904-01-01), timestamp(3682565790.191844 s since 1904-01-01), timestamp(3682565791.191016 s since 1904-01-01), timestamp(3682565792.191493 s since 1904-01-01), timestamp(3682565793.190962 s since 1904-01-01), timestamp(3682565794.192923 s since 1904-01-01), timestamp(3682565795.1943216 s since 1904-01-01), timestamp(3682565796.1945167 s since 1904-01-01), timestamp(3682565797.194023 s since 1904-01-01), timestamp(3682565798.1947985 s since 1904-01-01), timestamp(3682565799.194545 s since 1904-01-01), timestamp(3682565800.194017 s since 1904-01-01), timestamp(3682565801.1955366 s since 1904-01-01), timestamp(3682565802.1962314 s since 1904-01-01), timestamp(3682565803.1960993 s since 1904-01-01), timestamp(3682565804.196091 s since 1904-01-01), timestamp(3682565805.197301 s since 1904-01-01)], "DataArray"=[296.503, 296.505, 296.513, 296.51, 296.5, 296.502, 296.508, 296.503, 296.527, 296.517, 296.523, 296.514, 296.496, 296.516, 296.511, 296.521, 296.502, 296.504]}] caption="XY Graph"
  out "Graph 3":T8(graph)=[{"TimeArray"=[timestamp(3682565788.1889906 s since 1904-01-01), timestamp(3682565789.190164 s since 1904-01-01), timestamp(3682565790.191844 s since 1904-01-01), timestamp(3682565791.191016 s since 1904-01-01), timestamp(3682565792.191493 s since 1904-01-01), timestamp(3682565793.190962 s since 1904-01-01), timestamp(3682565794.192923 s since 1904-01-01), timestamp(3682565795.1943216 s since 1904-01-01), timestamp(3682565796.1945167 s since 1904-01-01), timestamp(3682565797.194023 s since 1904-01-01), timestamp(3682565798.195678 s since 1904-01-01), timestamp(3682565799.194545 s since 1904-01-01), timestamp(3682565800.194017 s since 1904-01-01), timestamp(3682565801.196416 s since 1904-01-01), timestamp(3682565802.1962314 s since 1904-01-01), timestamp(3682565803.1960993 s since 1904-01-01), timestamp(3682565804.196091 s since 1904-01-01), timestamp(3682565805.197301 s since 1904-01-01)], "DataArray"=[0.000981756523507472]}, {"TimeArray"=[timestamp(3682565788.1889906 s since 1904-01-01), timestamp(3682565789.190164 s since 1904-01-01), timestamp(3682565790.191844 s since 1904-01-01), timestamp(3682565791.191016 s since 1904-01-01), timestamp(3682565792.191493 s since 1904-01-01), timestamp(3682565793.190962 s since 1904-01-01), timestamp(3682565794.192923 s since 1904-01-01), timestamp(3682565795.1943216 s since 1904-01-01), timestamp(3682565796.1945167 s since 1904-01-01), timestamp(3682565797.194023 s since 1904-01-01), timestamp(3682565798.195678 s since 1904-01-01), timestamp(3682565799.194545 s since 1904-01-01), timestamp(3682565800.194017 s since 1904-01-01), timestamp(3682565801.196416 s since 1904-01-01), timestamp(3682565802.1962314 s since 1904-01-01), timestamp(3682565803.1960993 s since 1904-01-01), timestamp(3682565804.196091 s since 1904-01-01), timestamp(3682565805.197301 s since 1904-01-01)], "DataArray"=[101282.93029464335]}, {"TimeArray"=[timestamp(3682565788.1889906 s since 1904-01-01), timestamp(3682565789.190164 s since 1904-01-01), timestamp(3682565790.191844 s since 1904-01-01), timestamp(3682565791.191016 s since 1904-01-01), timestamp(3682565792.191493 s since 1904-01-01), timestamp(3682565793.190962 s since 1904-01-01), timestamp(3682565794.192923 s since 1904-01-01), timestamp(3682565795.1943216 s since 1904-01-01), timestamp(3682565796.1945167 s since 1904-01-01), timestamp(3682565797.194023 s since 1904-01-01), timestamp(3682565798.195678 s since 1904-01-01), timestamp(3682565799.194545 s since 1904-01-01), timestamp(3682565800.194017 s since 1904-01-01), timestamp(3682565801.196416 s since 1904-01-01), timestamp(3682565802.1962314 s since 1904-01-01), timestamp(3682565803.1960993 s since 1904-01-01), timestamp(3682565804.196091 s since 1904-01-01), timestamp(3682565805.197301 s since 1904-01-01)], "DataArray"=[100447.56177003749]}, {"TimeArray"=[timestamp(3682565788.1889906 s since 1904-01-01), timestamp(3682565789.190164 s since 1904-01-01), timestamp(3682565790.191844 s since 1904-01-01), timestamp(3682565791.191016 s since 1904-01-01), timestamp(3682565792.191493 s since 1904-01-01), timestamp(3682565793.190962 s since 1904-01-01), timestamp(3682565794.192923 s since 1904-01-01), timestamp(3682565795.1943216 s since 1904-01-01), timestamp(3682565796.1945167 s since 1904-01-01), timestamp(3682565797.194023 s since 1904-01-01), timestamp(3682565798.195678 s since 1904-01-01), timestamp(3682565799.194545 s since 1904-01-01), timestamp(3682565800.194017 s since 1904-01-01), timestamp(3682565801.196416 s since 1904-01-01), timestamp(3682565802.1962314 s since 1904-01-01), timestamp(3682565803.1960993 s since 1904-01-01), timestamp(3682565804.196091 s since 1904-01-01), timestamp(3682565805.197301 s since 1904-01-01)], "DataArray"=[100215.69769894995]}, {"TimeArray"=[timestamp(3682565788.1889906 s since 1904-01-01), timestamp(3682565789.190164 s since 1904-01-01), timestamp(3682565790.191844 s since 1904-01-01), timestamp(3682565791.191016 s since 1904-01-01), timestamp(3682565792.191493 s since 1904-01-01), timestamp(3682565793.190962 s since 1904-01-01), timestamp(3682565794.192923 s since 1904-01-01), timestamp(3682565795.1943216 s since 1904-01-01), timestamp(3682565796.1945167 s since 1904-01-01), timestamp(3682565797.194023 s since 1904-01-01), timestamp(3682565798.195678 s since 1904-01-01), timestamp(3682565799.194545 s since 1904-01-01), timestamp(3682565800.194017 s since 1904-01-01), timestamp(3682565801.196416 s since 1904-01-01), timestamp(3682565802.1962314 s since 1904-01-01), timestamp(3682565803.1960993 s since 1904-01-01), timestamp(3682565804.196091 s since 1904-01-01), timestamp(3682565805.197301 s since 1904-01-01)], "DataArray"=[100421.61018172985]}, {"TimeArray"=[timestamp(3682565788.1889906 s since 1904-01-01), timestamp(3682565789.190164 s since 1904-01-01), timestamp(3682565790.191844 s since 1904-01-01), timestamp(3682565791.191016 s since 1904-01-01), timestamp(3682565792.191493 s since 1904-01-01), timestamp(3682565793.190962 s since 1904-01-01), timestamp(3682565794.192923 s since 1904-01-01), timestamp(3682565795.1943216 s since 1904-01-01), timestamp(3682565796.1945167 s since 1904-01-01), timestamp(3682565797.194023 s since 1904-01-01), timestamp(3682565798.195678 s since 1904-01-01), timestamp(3682565799.194545 s since 1904-01-01), timestamp(3682565800.194017 s since 1904-01-01), timestamp(3682565801.196416 s since 1904-01-01), timestamp(3682565802.1962314 s since 1904-01-01), timestamp(3682565803.1960993 s since 1904-01-01), timestamp(3682565804.196091 s since 1904-01-01), timestamp(3682565805.197301 s since 1904-01-01)], "DataArray"=[100780.20754019849]}, {"TimeArray"=[timestamp(3682565788.1889906 s since 1904-01-01), timestamp(3682565789.190164 s since 1904-01-01), timestamp(3682565790.191844 s since 1904-01-01), timestamp(3682565791.191016 s since 1904-01-01), timestamp(3682565792.191493 s since 1904-01-01), timestamp(3682565793.190962 s since 1904-01-01), timestamp(3682565794.192923 s since 1904-01-01), timestamp(3682565795.1943216 s since 1904-01-01), timestamp(3682565796.1945167 s since 1904-01-01), timestamp(3682565797.194023 s since 1904-01-01), timestamp(3682565798.195678 s since 1904-01-01), timestamp(3682565799.194545 s since 1904-01-01), timestamp(3682565800.194017 s since 1904-01-01), timestamp(3682565801.196416 s since 1904-01-01), timestamp(3682565802.1962314 s since 1904-01-01), timestamp(3682565803.1960993 s since 1904-01-01), timestamp(3682565804.196091 s since 1904-01-01), timestamp(3682565805.197301 s since 1904-01-01)], "DataArray"=[-9.626849444535207]}, {"TimeArray"=[timestamp(3682565788.1889906 s since 1904-01-01), timestamp(3682565789.190164 s since 1904-01-01), timestamp(3682565790.191844 s since 1904-01-01), timestamp(3682565791.191016 s since 1904-01-01), timestamp(3682565792.191493 s since 1904-01-01), timestamp(3682565793.190962 s since 1904-01-01), timestamp(3682565794.192923 s since 1904-01-01), timestamp(3682565795.1943216 s since 1904-01-01), timestamp(3682565796.1945167 s since 1904-01-01), timestamp(3682565797.194023 s since 1904-01-01), timestamp(3682565798.195678 s since 1904-01-01), timestamp(3682565799.194545 s since 1904-01-01), timestamp(3682565800.194017 s since 1904-01-01), timestamp(3682565801.196416 s since 1904-01-01), timestamp(3682565802.1962314 s since 1904-01-01), timestamp(3682565803.1960993 s since 1904-01-01), timestamp(3682565804.196091 s since 1904-01-01), timestamp(3682565805.197301 s since 1904-01-01)], "DataArray"=[78.6252889928285]}] caption="XY Graph"
  out "Graph 4":T8(graph)=[{"TimeArray"=[timestamp(3682565788.1889906 s since 1904-01-01), timestamp(3682565789.190164 s since 1904-01-01), timestamp(3682565790.191844 s since 1904-01-01), timestamp(3682565791.191016 s since 1904-01-01), timestamp(3682565792.191493 s since 1904-01-01), timestamp(3682565793.190962 s since 1904-01-01), timestamp(3682565794.192923 s since 1904-01-01), timestamp(3682565795.1943216 s since 1904-01-01), timestamp(3682565796.1945167 s since 1904-01-01), timestamp(3682565797.194023 s since 1904-01-01), timestamp(3682565798.195678 s since 1904-01-01), timestamp(3682565799.194545 s since 1904-01-01), timestamp(3682565800.194017 s since 1904-01-01), timestamp(3682565801.196416 s since 1904-01-01), timestamp(3682565802.1962314 s since 1904-01-01), timestamp(3682565803.1960993 s since 1904-01-01), timestamp(3682565804.196091 s since 1904-01-01), timestamp(3682565805.197301 s since 1904-01-01)], "DataArray"=[100.08609659349952]}, {"TimeArray"=[timestamp(3682565788.1889906 s since 1904-01-01), timestamp(3682565789.190164 s since 1904-01-01), timestamp(3682565790.191844 s since 1904-01-01), timestamp(3682565791.191016 s since 1904-01-01), timestamp(3682565792.191493 s since 1904-01-01), timestamp(3682565793.190962 s since 1904-01-01), timestamp(3682565794.192923 s since 1904-01-01), timestamp(3682565795.1943216 s since 1904-01-01), timestamp(3682565796.1945167 s since 1904-01-01), timestamp(3682565797.194023 s since 1904-01-01), timestamp(3682565798.195678 s since 1904-01-01), timestamp(3682565799.194545 s since 1904-01-01), timestamp(3682565800.194017 s since 1904-01-01), timestamp(3682565801.196416 s since 1904-01-01), timestamp(3682565802.1962314 s since 1904-01-01), timestamp(3682565803.1960993 s since 1904-01-01), timestamp(3682565804.196091 s since 1904-01-01), timestamp(3682565805.197301 s since 1904-01-01)], "DataArray"=[0.1296859810079549]}, {"TimeArray"=[timestamp(3682565788.1889906 s since 1904-01-01), timestamp(3682565789.190164 s since 1904-01-01), timestamp(3682565790.191844 s since 1904-01-01), timestamp(3682565791.191016 s since 1904-01-01), timestamp(3682565792.191493 s since 1904-01-01), timestamp(3682565793.190962 s since 1904-01-01), timestamp(3682565794.192923 s since 1904-01-01), timestamp(3682565795.1943216 s since 1904-01-01), timestamp(3682565796.1945167 s since 1904-01-01), timestamp(3682565797.194023 s since 1904-01-01), timestamp(3682565798.195678 s since 1904-01-01), timestamp(3682565799.194545 s since 1904-01-01), timestamp(3682565800.194017 s since 1904-01-01), timestamp(3682565801.196416 s since 1904-01-01), timestamp(3682565802.1962314 s since 1904-01-01), timestamp(3682565803.1960993 s since 1904-01-01), timestamp(3682565804.196091 s since 1904-01-01), timestamp(3682565805.197301 s since 1904-01-01)], "DataArray"=[0.1356046075893618]}, {"TimeArray"=[timestamp(3682565788.1889906 s since 1904-01-01), timestamp(3682565789.190164 s since 1904-01-01), timestamp(3682565790.191844 s since 1904-01-01), timestamp(3682565791.191016 s since 1904-01-01), timestamp(3682565792.191493 